vi "Experiment_ANTENNA_RADIATION.vi"() -> ()   [LabVIEW 2009]
uses:
  <vilib>/imath/engines/lvmath2/RunTimeEngine/ErrorHandling/NIMS_Finalize Error.vi
  <vilib>/imath/engines/lvmath2/RunTimeEngine/Parser/MC_Version.vi
  <vilib>/imath/engines/lvmath2/RunTimeEngine/Managers/WorkSpace/UID Generator.vi
  <vilib>/imath/engines/lvmath2/RunTimeEngine/NodeEndStatement/NIMS_NodeEndStatement_Output.vi
  <instcachedir>/0/NIMS_NodeEndStatement_Output_B70DDD75627E4997AAE11E9955EDAA25.lvgen/NIMS_NodeEndStatement_Output_B70DDD75627E4997AAE11E9955EDAA25_001.vi
  <vilib>/imath/engines/lvmath2/RunTimeEngine/Managers/SymbolTable/Clear UID.vi
  <vilib>/imath/engines/lvmath2/RunTimeEngine/LocalVariableDefStatement/MC_LocalVariableDefStatement_Display.vi
  <vilib>/imath/engines/lvmath2/RunTimeEngine/RunTimeType/NIMS_RunTimeType_From StrictType (excl LVString).vi
  <vilib>/imath/engines/lvmath2/RunTimeEngine/RangeToken/NIMS_Range.vi
  <instcachedir>/0/NIMS_Range_6D647EC16A744C98B5DE1D649A2D648D.lvgen/NIMS_Range_6D647EC16A744C98B5DE1D649A2D648D_001.vi
  <vilib>/imath/engines/lvmath/Functions/Error Handling/error.ctl
  <vilib>/imath/engines/lvmath/Functions/Error Handling/MergeErrorsWrapper.vi
  <vilib>/imath/engines/lvmath2/RunTimeEngine/VariableToken/NIMS_VariableToken_CondDefined.vi
  <instcachedir>/0/NIMS_VariableToken_CondDefined_5641E79000FB4D628475532441475385.lvgen/NIMS_VariableToken_CondDefined_5641E79000FB4D628475532441475385_002.vi
  <vilib>/imath/engines/lvmath/Functions/Error Handling/MC_Mask_Errors.vi
  <vilib>/imath/engines/lvmath2/RunTimeEngine/BuiltInFunctions/rem/NIMS_rem_no checks.vi
  <instcachedir>/0/NIMS_rem_no checks_4CC9B305AB7E42EF90AFC4973FB32F8D.lvgen/NIMS_rem_no checks_4CC9B305AB7E42EF90AFC4973FB32F8D_000.vi
  <vilib>/imath/engines/lvmath2/RunTimeEngine/BuiltInFunctions/uint32/NIMS_uint32(real).vi
  <instcachedir>/0/NIMS_uint32(real)_FDC83D68D45943DDB8F3F934FF8A712F.lvgen/NIMS_uint32(real)_FDC83D68D45943DDB8F3F934FF8A712F_000.vi
  <vilib>/imath/engines/lvmath2/RunTimeEngine/BuiltInFunctions/double/NIMS_double.vi
  <instcachedir>/0/NIMS_double_2CE444F3CE4146B199A482FE12545E45.lvgen/NIMS_double_2CE444F3CE4146B199A482FE12545E45_000.vi
  <vilib>/imath/engines/lvmath2/RunTimeEngine/BuiltInFunctions/length/NIMS_length(GV).vi
  <instcachedir>/0/NIMS_length(GV)_7D6E94E728E145E68721C53861296D96.lvgen/NIMS_length(GV)_7D6E94E728E145E68721C53861296D96_000.vi
  <instcachedir>/0/NIMS_Range_6D647EC16A744C98B5DE1D649A2D648D.lvgen/NIMS_Range_6D647EC16A744C98B5DE1D649A2D648D_000.vi
  <vilib>/imathl/engines/lvmath/Functions/Error Handling/Create Error.vi
  <vilib>/imath/engines/lvmath2/RunTimeEngine/ReplaceToken/NIMS_Replace - V(S)=S.vi
  <instcachedir>/0/NIMS_Replace - V(S)=S_670A9E0533664C1D848C8E58B3321B6A.lvgen/NIMS_Replace - V(S)=S_670A9E0533664C1D848C8E58B3321B6A_001.vi
  <vilib>/imath/engines/lvmath2/RunTimeEngine/ReplaceToken/NIMS_Replace - Size Check _(_)=S.vi
  <instcachedir>/0/NIMS_Replace - Size Check _(_)=S_8596181D73404097BAB9CBB006194BB0.lvgen/NIMS_Replace - Size Check _(_)=S_8596181D73404097BAB9CBB006194BB0_002.vi
  <vilib>/imath/engines/lvmath2/RunTimeEngine/ReplaceToken/NIMS_Replace - Check Linear.vi
  <instcachedir>/0/NIMS_Replace - Check Linear_9243CBB174894FF6977027453DA6955E.lvgen/NIMS_Replace - Check Linear_9243CBB174894FF6977027453DA6955E_002.vi
  <vilib>/imath/engines/lvmath2/RunTimeEngine/VariableToken/NIMS_VariableToken_CondDefinedDefinedByReplace.vi
  <instcachedir>/0/NIMS_VariableToken_CondDefinedDefinedByReplace_D162CFFC24174562A9FEA619A91E1A56.lvgen/NIMS_VariableToken_CondDefinedDefinedByReplace_D162CFFC24174562A9FEA619A91E1A56_002.vi
  <vilib>/imath/engines/lvmath2/RunTimeEngine/CommandStatement/MC_CommandStatement_break.vi
  <vilib>/imath/engines/lvmath2/RunTimeEngine/ArithmeticOperatorToken/NIMS_ArithmeticOperator_times.vi
  <instcachedir>/0/NIMS_ArithmeticOperator_times_3987BC660D7947CD8628C10658A43225.lvgen/NIMS_ArithmeticOperator_times_3987BC660D7947CD8628C10658A43225_001.vi
  <instcachedir>/0/NIMS_NodeEndStatement_Output_B70DDD75627E4997AAE11E9955EDAA25.lvgen/NIMS_NodeEndStatement_Output_B70DDD75627E4997AAE11E9955EDAA25_000.vi
  <instcachedir>/0/NIMS_ArithmeticOperator_times_3987BC660D7947CD8628C10658A43225.lvgen/NIMS_ArithmeticOperator_times_3987BC660D7947CD8628C10658A43225_000.vi
  <vilib>/imath/engines/lvmath2/RunTimeEngine/VariableToken/Read/NIMS_Get Elements - RV(_) - Check.vi
  <instcachedir>/0/NIMS_Get Elements - RV(_) - Check_60F12861D0564803969A5D0D0D1716CD.lvgen/NIMS_Get Elements - RV(_) - Check_60F12861D0564803969A5D0D0D1716CD_001.vi
  <vilib>/imath/engines/lvmath2/RunTimeEngine/BuiltInFunctions/abs/NIMS_abs(signed).vi
  <instcachedir>/0/NIMS_abs(signed)_C4FCB8E6058B49B797C7C8D53CA5F6EC.lvgen/NIMS_abs(signed)_C4FCB8E6058B49B797C7C8D53CA5F6EC_000.vi
  <instcachedir>/0/NIMS_VariableToken_CondDefined_5641E79000FB4D628475532441475385.lvgen/NIMS_VariableToken_CondDefined_5641E79000FB4D628475532441475385_003.vi
  <instcachedir>/0/NIMS_Replace - V(S)=S_670A9E0533664C1D848C8E58B3321B6A.lvgen/NIMS_Replace - V(S)=S_670A9E0533664C1D848C8E58B3321B6A_000.vi
  <instcachedir>/0/NIMS_Replace - Size Check _(_)=S_8596181D73404097BAB9CBB006194BB0.lvgen/NIMS_Replace - Size Check _(_)=S_8596181D73404097BAB9CBB006194BB0_001.vi
  <instcachedir>/0/NIMS_Replace - Check Linear_9243CBB174894FF6977027453DA6955E.lvgen/NIMS_Replace - Check Linear_9243CBB174894FF6977027453DA6955E_001.vi
  <instcachedir>/0/NIMS_VariableToken_CondDefinedDefinedByReplace_D162CFFC24174562A9FEA619A91E1A56.lvgen/NIMS_VariableToken_CondDefinedDefinedByReplace_D162CFFC24174562A9FEA619A91E1A56_001.vi
  <instcachedir>/0/NIMS_VariableToken_CondDefined_5641E79000FB4D628475532441475385.lvgen/NIMS_VariableToken_CondDefined_5641E79000FB4D628475532441475385_001.vi
  <instcachedir>/0/NIMS_Replace - V(S)=S_670A9E0533664C1D848C8E58B3321B6A.lvgen/NIMS_Replace - V(S)=S_670A9E0533664C1D848C8E58B3321B6A_002.vi
  <instcachedir>/0/NIMS_Replace - Size Check _(_)=S_8596181D73404097BAB9CBB006194BB0.lvgen/NIMS_Replace - Size Check _(_)=S_8596181D73404097BAB9CBB006194BB0_003.vi
  <instcachedir>/0/NIMS_Replace - Check Linear_9243CBB174894FF6977027453DA6955E.lvgen/NIMS_Replace - Check Linear_9243CBB174894FF6977027453DA6955E_003.vi
  <instcachedir>/0/NIMS_VariableToken_CondDefinedDefinedByReplace_D162CFFC24174562A9FEA619A91E1A56.lvgen/NIMS_VariableToken_CondDefinedDefinedByReplace_D162CFFC24174562A9FEA619A91E1A56_003.vi
  <vilib>/gmath/NI_Gmath.lvlib
  <vilib>/imath/engines/lvmath2/RunTimeEngine/Managers/SymbolTable/NIMS_WorkSpace.lvlib
panel:
  out "error out":errorcluster
  in  "?":T1(tab)
  out "?":cluster{"Y":dbl[], "Y":dbl[]}[](graph)
  in  "HELP FOR FIELD PATTERN":bool
  out "?":cluster{"Y":dbl[], "Y":dbl[]}[](graph)
  in  "?":enum32{"ATTENUATOR"}(tab)
  out "?":dbl[](graph)
  in  "Set the value of attenuation in dB":dbl(slide) scale=0.0..100.0
  out "?":errorcluster
  in  "HELP FOR ATTENUATOR":bool
  out "error out":errorcluster
  in  "?":enum32{"ISOLATOR"}(tab)
  out "?":dbl[](graph)
  in  "?":bool
  out "?":errorcluster
  in  "HELP FOR ISOLATOR":bool
  out "error out":errorcluster
  in  "?":enum32{"MODULATOR"}(tab)
  in  "Modulating Frequency(KHz)":dbl(slide) scale=0.5..1.5
  out "?":errorcluster
  out "?":dbl[](graph)
  in  "HELP FOR MODULATOR":bool
  out "error out":errorcluster
  in  "?":enum32{"SOURCE"}(tab)
  out "?":dbl[](graph)
  in  "Frequency of carrier wave(GHz)":dbl(slide) scale=8.0..15.0
  in  "Voltage":dbl(knob) scale=0.0..20.0 scale format="%#_10g"
  out "?":errorcluster
  in  "HELP FOR SOURCE":bool
  out "error out":errorcluster
  # "Source"
  # "Variable Attenuator"
  # "Trasmittind and Receiving Antenna"
  # "VSWR Meter"
  # "Coaxial to rectangular adapter"
  # "Connecting waveguide"
  # "Isolator"
  # "Connecting waveguide"
  # "Backward Direction"
  # "Forward direction"
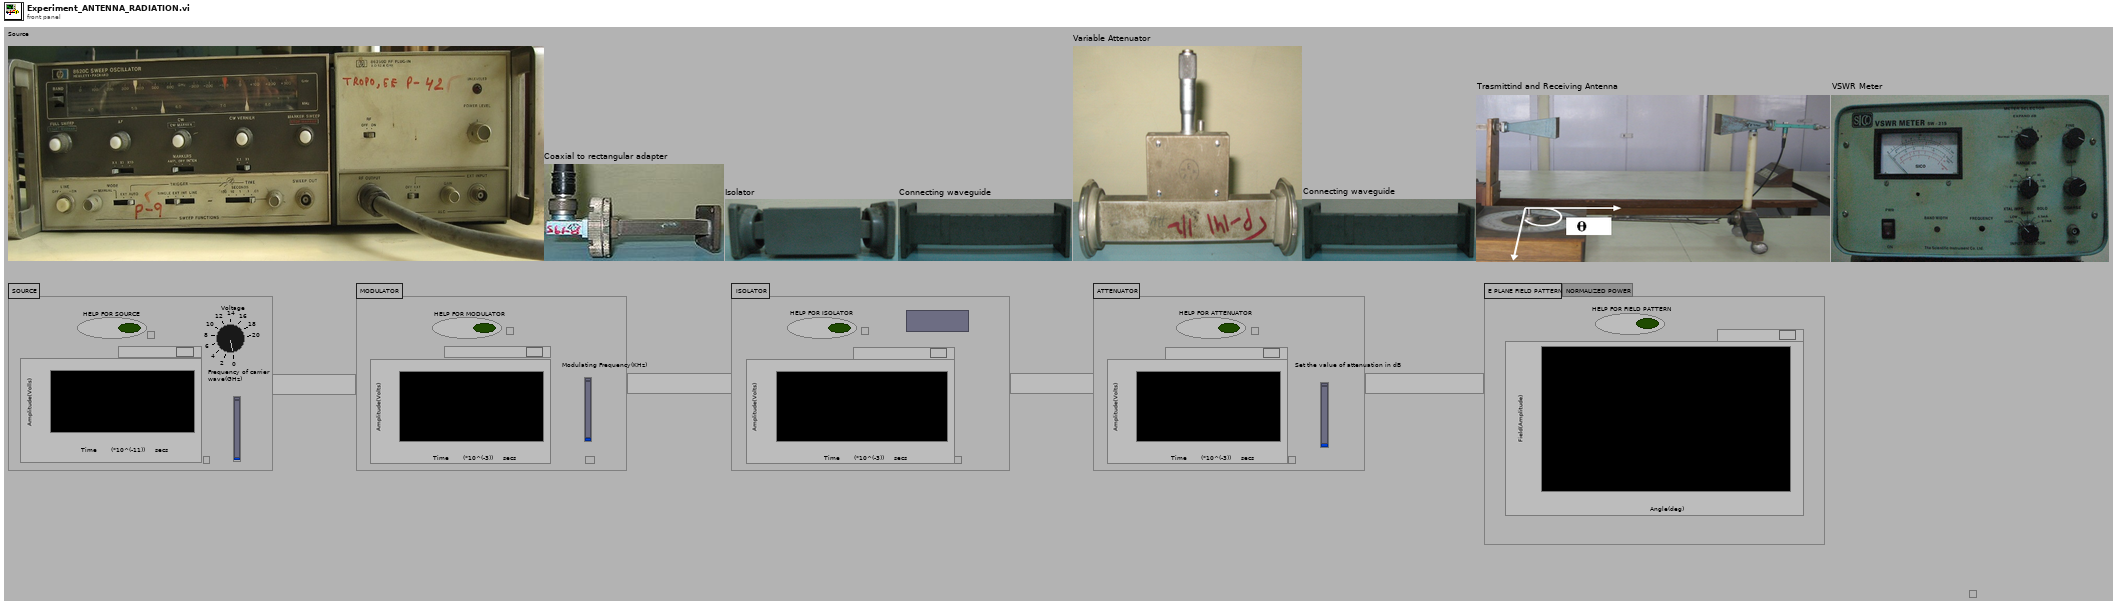
[diagram p1: front panel]
types:
  T1 = enum32{"E PLANE FIELD PATTERN", "NORMALIZED POWER"}
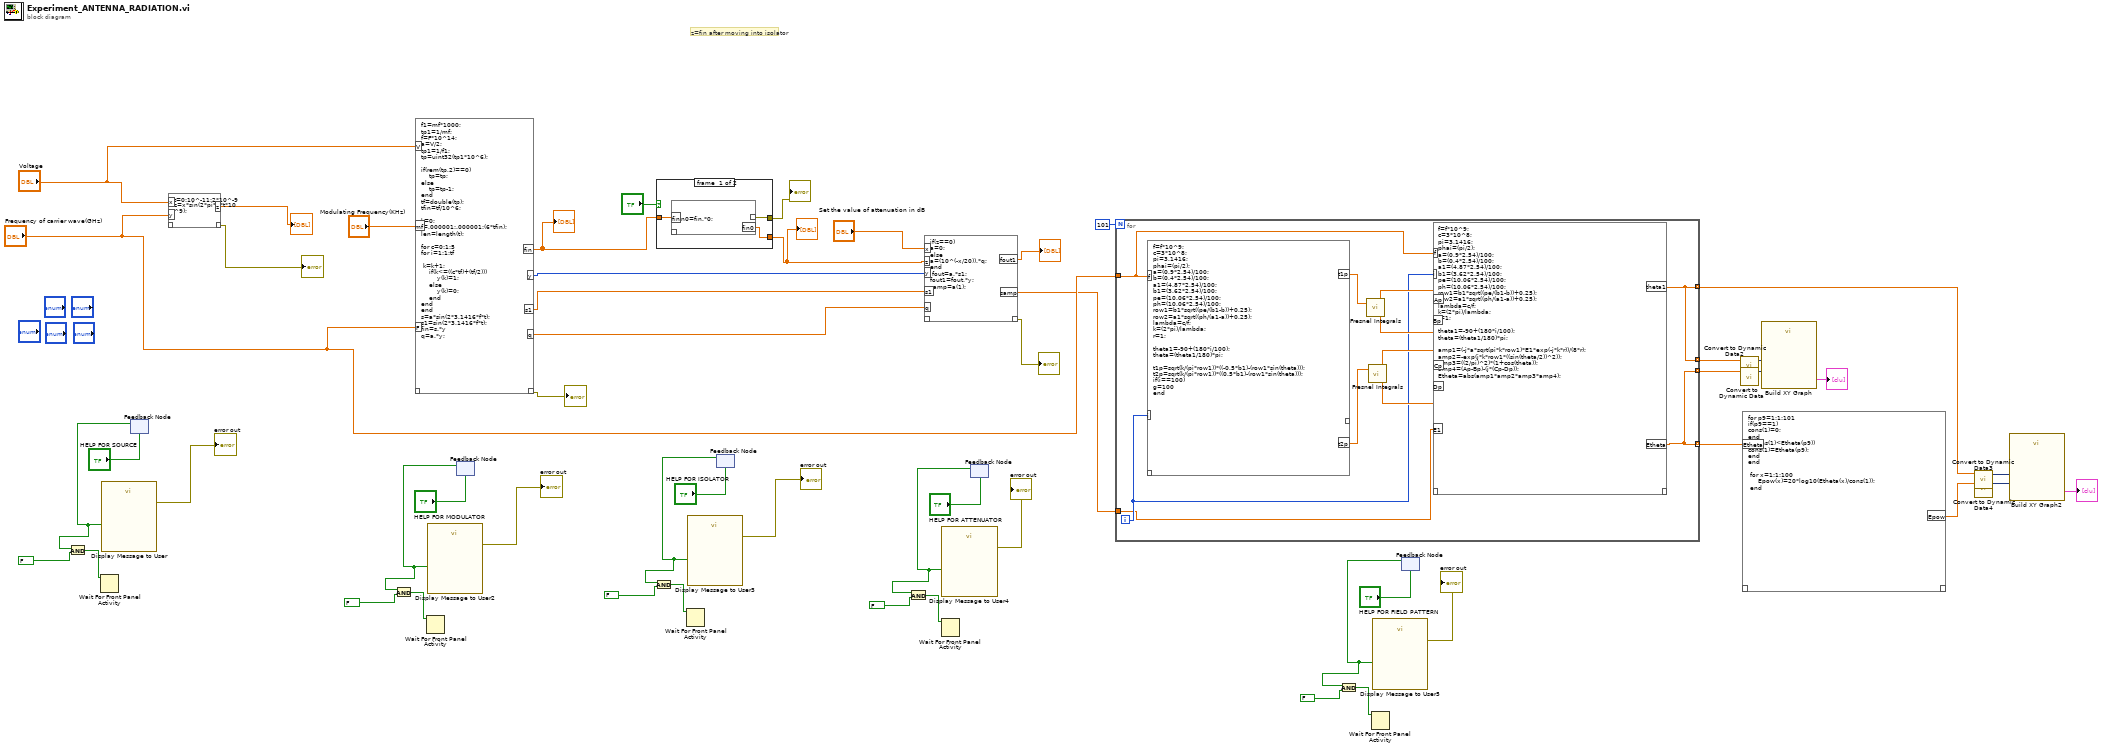
[diagram p0: block diagram]
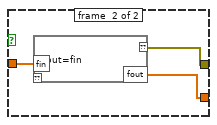
[diagram p2: hidden frame]
diagram:
  # "z=fin after moving into isolator"
  n1 = feedback #1("HELP FOR SOURCE") -> (w54:bool)
  n2 = And(x=w54, y=FALSE) -> (x .and. y?=w52:bool)
  n3 = Wait For Front Panel Activity(3:w52) -> ()  [unwired: 3 out]
  n4 = call "Display Message to User"("Enable"=w54) -> ("error out"=→"error out":errorcluster, "CLOSE"=w56:bool)  [unwired: 2 in, 7 out]
  n5 = mathscript code="t=0:10^-11:2*10^-9\nz=x*sin(2*pi*y*t*10^9);"("x"="Voltage", "y"="Frequency of carrier wave(GHz)") -> ("??"=→"?":errorcluster, "z"=→"?":dbl[])  [unwired: 1 in]
  n6 = mathscript code="f1=mf*1000;\ntp1=1/mf;\nf=F*10^14;\na=V/2;\ntp1=1/f1;\ntp=uint32(tp1*10^6);\n\nif(rem(tp,2)==0)\n    tp=tp;\nelse\n    tp=tp-1;\nend\ntf=double(tp);\ntfin=tf/10^6;\n\nk=0;\nt=.000001:.000001:(6*tfin);\nlen=length(t);\n\nfor c=0:1:5\nfor i=1:1:tf\n  \n k=k+1;\n    if(k<=((c*tf)+(tf/2)))\n        y(k)=1;\n    else\n        y(k)=0;\n    end\nend\nend\ns=a*sin(2*3.1416*f*t);\ns1=sin(2*3.1416*f*t);\nfin=s.*y\nq=a.*y;"("V"="Voltage", "mf"="Modulating Frequency(KHz)", "F"="Frequency of carrier wave(GHz)") -> ("??"=→"?":errorcluster, "y"=w11:i32[], "s1"=w18:dbl[], "q"=w17:dbl[], "fin"=w10:dbl[])  [unwired: 1 in]
  "?" <- w10
  n7 = feedback #2("HELP FOR MODULATOR") -> (w48:bool)
  n8 = And(x=w48, y=FALSE) -> (x .and. y?=w46:bool)
  n9 = Wait For Front Panel Activity(3:w46) -> ()  [unwired: 3 out]
  n10 = call "Display Message to User2"("Enable"=w48) -> ("error out"=→"error out":errorcluster, "CLOSE"=w50:bool)  [unwired: 2 in, 7 out]
  n11 = case shown="True" "?" {
    tunnel: [w61 w82] -> w9
    tunnel: [w62 w83] -> w58
    tunnel: w10 -> [w60 w81]
    frame #0 {
      n12 = mathscript code="fin0=fin.*0;"("fin"=w60) -> ("??"=w62:errorcluster, "fin0"=w61:dbl[])  [unwired: 1 in]
    }
    frame #1 {
      n13 = mathscript code="fout=fin"("fin"=w81) -> ("??"=w83:errorcluster, "fout"=w82:dbl[])  [unwired: 1 in]
    }
  }
  "?" <- w9
  "?" <- w58
  n14 = feedback #3("HELP FOR ISOLATOR") -> (w42:bool)
  n15 = And(x=w42, y=FALSE) -> (x .and. y?=w40:bool)
  n16 = Wait For Front Panel Activity(3:w40) -> ()  [unwired: 3 out]
  n17 = call "Display Message to User3"("Enable"=w42) -> ("error out"=→"error out":errorcluster, "CLOSE"=w44:bool)  [unwired: 2 in, 7 out]
  n18 = mathscript code="if(z==0)\na=0; \nelse\na=(10^(-x/20)).*q;\nend\n fout=a.*s1;\nfout1=fout.*y;\nsamp=a(1);"("x"="Set the value of attenuation in dB", "z"=w9, "y"=w11, "s1"=w18, "q"=w17) -> ("??"=→"?":errorcluster, "fout1"=→"?":dbl[], "samp"=w12:dbl)  [unwired: 1 in]
  n19 = feedback #4("HELP FOR ATTENUATOR") -> (w36:bool)
  n20 = And(x=w36, y=FALSE) -> (x .and. y?=w34:bool)
  n21 = Wait For Front Panel Activity(3:w34) -> ()  [unwired: 3 out]
  n22 = call "Display Message to User4"("Enable"=w36) -> ("error out"=→"error out":errorcluster, "CLOSE"=w38:bool)  [unwired: 2 in, 7 out]
  n23 = for {
    N: 101 -> [_]
    tunnel: "Frequency of carrier wave(GHz)" -> [w119]
    tunnel: [w116] -> w30 mode=indexing
    tunnel: [w118] -> w28 mode=indexing
    tunnel: [w116] -> w26 mode=indexing
    tunnel: [w118] -> w25 mode=indexing
    tunnel: w12 -> [w117]
    i -> [w120]
    n24 = mathscript code="f=f*10^9;\nc=3*10^8;\npi=3.1416;\nphai=(pi/2);\na=(0.9*2.54)/100;\nb=(0.4*2.54)/100;\na1=(4.87*2.54)/100;\nb1=(3.62*2.54)/100;\npe=(10.06*2.54)/100;\nph=(10.06*2.54)/100;\nrow1=b1*sqrt((pe/(b1-b))+0.25);\nrow2=a1*sqrt((ph/(a1-a))+0.25);\nlambda=c/f;\nk=(2*pi)/lambda;\nr=1;\n\ntheta1=-90+(180*i/100);\ntheta=(theta1/180)*pi;\n   \nt1p=sqrt(k/(pi*row1))*((-0.5*b1)-(row1*sin(theta)));\nt2p=sqrt(k/(pi*row1))*((0.5*b1)-(row1*sin(theta)));\nif(i==100)\ng=100\nend"("i"=w120, "f"=w119) -> ("t1p"=w126:dbl, "t2p"=w125:dbl)  [unwired: 2 out]
    n25 = call <vilib>:"Fresnel Integrals.vi"("x"=w126) -> ("S(x)"=w121:dbl, "C(x)"=w123:dbl)  [unwired: 1 out]
    n26 = call <vilib>:"Fresnel Integrals.vi"("x"=w125) -> ("S(x)"=w122:dbl, "C(x)"=w124:dbl)  [unwired: 1 out]
    n27 = mathscript code="f=f*10^9;\nc=3*10^8;\npi=3.1416;\nphai=(pi/2);\na=(0.9*2.54)/100;\nb=(0.4*2.54)/100;\na1=(4.87*2.54)/100;\nb1=(3.62*2.54)/100;\npe=(10.06*2.54)/100;\nph=(10.06*2.54)/100;\nrow1=b1*sqrt((pe/(b1-b))+0.25);\nrow2=a1*sqrt((ph/(a1-a))+0.25);\nlambda=c/f;\nk=(2*pi)/lambda;\nr=1;\n \ntheta1=-90+(180*i/100);\ntheta=(theta1/180)*pi;\n    \namp1=(-j*a*sqrt(pi*k*row1)*E1*exp(-j*k*r))/(8*r);\namp2=-exp(j*k*row1*((sin(theta/2))^2));\namp3=((2/pi)^2)*(1+cos(theta));\namp4=(Ap-Bp)-(j*(Cp-Dp));\nEtheta=abs(amp1*amp2*amp3*amp4);"("Ap"=w124, "Bp"=w123, "Cp"=w122, "Dp"=w121, "i"=w120, "E1"=w117, "f"=w119) -> ("Etheta"=w116:dbl, "theta1"=w118:dbl)  [unwired: 2 out]
  }
  n28 = feedback #5("HELP FOR FIELD PATTERN") -> (w3:bool)
  n29 = And(x=w3, y=FALSE) -> (x .and. y?=w1:bool)
  n30 = Wait For Front Panel Activity(3:w1) -> ()  [unwired: 3 out]
  n31 = call "Display Message to User5"("Enable"=w3) -> ("error out"=→"error out":errorcluster, "CLOSE"=w5:bool)  [unwired: 2 in, 7 out]
  n32 = call "Convert to Dynamic Data2"("Array"=w28) -> ("Dynamic Data Type"=w27:dynamicdata)  [unwired: 3 out]
  n33 = call "Convert to Dynamic Data"("Array"=w30) -> ("Dynamic Data Type"=w29:dynamicdata)  [unwired: 3 out]
  n34 = mathscript code="for p9=1:1:101\nif(p9==1)\ncons(1)=0;\nend\nif(cons(1)<Etheta(p9))\ncons(1)=Etheta(p9);\nend\nend\n\n for x=1:1:100\n     Epow(x)=20*log10(Etheta(x)/cons(1));\n end"("Etheta"=w26) -> ("Epow"=w23:dbl[])  [unwired: 2 out]
  n35 = call "Build XY Graph"("Y Input"=w29, "X Input"=w27) -> ("XY Graph"=→"?":cluster{"Y":dbl[], "Y":dbl[]}[])  [unwired: 3 in, 6 out]
  n36 = call "Convert to Dynamic Data3"("Array"=w25) -> ("Dynamic Data Type"=w24:dynamicdata)  [unwired: 3 out]
  n37 = call "Convert to Dynamic Data4"("Array"=w23) -> ("Dynamic Data Type"=w22:dynamicdata)  [unwired: 3 out]
  n38 = call "Build XY Graph2"("Y Input"=w22, "X Input"=w24) -> ("XY Graph"=→"?":cluster{"Y":dbl[], "Y":dbl[]}[])  [unwired: 3 in, 6 out]
